vi "UHR-Fleezers Control (host) - Avogadro v3.vi"() -> ()   [LabVIEW 2014] (continued)
  out "Fluorescence laser intensities plot":cluster{dbl, dbl, dbl}(graph)
  in  "Green FB On/Off":bool
  in  "Red FB On/Off":bool
  in  "Blue FB On/Off":bool
  in  "Red Intensity % (FB OFF)":dbl=20.0 min=0.0 max=100.0 step=1.0
  in  "Blue Intensity % (FB OFF)":dbl=87.0 min=0.0 max=100.0 step=1.0
  out "Green laser intensity (V)":dbl
  in  "Initial Phase Adjustment (Green FB)":i16=-30
  in  "Phase adj. (Green FB)":i16=10
  out "Green AI Count":u16=600
  in  "- phase (Green FB)":bool
  in  "+ phase (Green FB)":bool
  out "Relative phase (Green FB)":i16
  out "GI Late Counter 2":u8
  in  "Phase adj. (GI) 2":i16=1
  out "GI relative phase 2":i16
  in  "+ phase (GI) 2":bool
  in  "Initial Phase Adjustment (GI) 2":i16=-274
  in  "- phase (GI) 2":bool
  in  "Green FB Gains":T18={"proportional gain (Kc)"=10, "integral gain (Kc*Ts/Ti)"=5, "derivative gain (Kc*Td/Ts)"=0}
  in  "Green int current ON count adj":u32=150
  out "Green AI Late Counter":u8
  out "MCL Scan":cluster{"Begin (V)":dbl, dbl, dbl[]}(graph)
  out "MCL Scan 2":cluster{"Begin (V)":dbl, dbl, dbl[]}(graph)
  out "Red laser intensity (V)":dbl
  out "Red AI Count":u16=600
  in  "Initial Phase Adjustment (RI)":i16=25
  out "RI Late Counter":u8
  in  "Red FB Gains":T18={"proportional gain (Kc)"=10, "integral gain (Kc*Ts/Ti)"=5, "derivative gain (Kc*Td/Ts)"=0}
  in  "Phase adj. (RI)":i16=20
  out "RI relative phase":i16
  in  "+ phase (RI)":bool
  in  "- phase (RI)":bool
  in  "Blue Laser Modulation Mode":string(combo)
  out "Digital Modulation":bool
  out "Analog Modulation":bool
  out "Laser On":bool
  in  "Get Blue Laser State":bool
  out "Blue laser intensity (V)":dbl
  out "Relative phase (BI AO)":i16
  out "Relative phase (BI DO)":i16
  out "Late Counter (BI DO)":u8
  out "Late Counter (BI AO)":u8
  in  "Initial Phase Adjustment (BI DO)":i16=65
  in  "Initial Phase Adjustment (BI AO)":i16
  in  "Phase adj. (BI AO)":i16=20
  in  "+ phase (BI AO)":bool
  in  "- phase (BI AO)":bool
  in  "Blue int AO ON count adjust":u16=150
  in  "Blue FB Gains":T18={"proportional gain (Kc)"=10, "integral gain (Kc*Ts/Ti)"=5, "derivative gain (Kc*Td/Ts)"=0}
  in  "- phase (BI DO)":bool
  in  "+ phase (BI DO)":bool
  in  "Phase adj. (BI DO)":i16=20
  out "Blue AI Count":u16=600
  in  "Delay (ms)":i32=500
  in  "Send string\nto Blue Laser":bool
  in  "command string":string
  out "command string sent":string="sames 0"
  out "read blue buffer":string
  out "Blue Error Out":errorcluster={"status"=TRUE, "code"=-1073807346, "source"="VISA Write in serial write macro.vi->UHR-Fleezers Control (host) - Avogadro v2.vi"}
  in  "VISA resource name":refnum<visa-resource-name>="Blue-Laser-COM7"
  in  "Blue Laser Modulation\nPower (mW)":string="80"
  in  "Blue Laser Power (mW)\n(Constant Power Mode)":string="70"
  in  "Laser choice 2":enum8{"Blue", "Green", "Red"}(ring)
  in  "Laser choice 1":enum8{"Blue", "Green", "Red"}(ring)
  in  "Laser choice 0":enum8{"Blue", "Green", "Red"}(ring)
  in  "FL interlace OFF count 2":u16=450
  in  "FL interlace OFF count 1":u16=450
  in  "FL interlace OFF count 0":u16=450
  in  "FL interlace ON count 2":u16=150
  in  "Fl interlace ON count 1":u16=150
  in  "FL interlace ON count 0":u16=150
  out "Vortran Late Counter":u8
  in  "Phase adj. (Vortran)":i16=1
  out "Vortran relative phase":i16
  in  "+ phase (Vortran)":bool
  in  "Initial Phase Adjustment (Vortran)":i16=-31
  in  "- phase (Vortran)":bool
  in  "Flip X Sign":bool=TRUE
  in  "Trap Position FIFO Depth":u32=500000 format="%.0p"
  in  "# Samples/trap":u32=20000
  out "Trap AI Elements/DMA read":u32=320000 format="%.0p"
  out "Ave. Rate (Hz)":dbl=200000.0 format="%#_6p"
  out "FIFO El. Rem.":u32=3 format="%.0p"
  in  "Phase adj. (AI1)":i16=10
  out "Relative phase (AI1)":i16=-186
  in  "+ phase (AI1)":bool
  in  "- phase (AI1)":bool
  out "Late Counter (AI1)":u8
  in  "Initial Phase Adjustment (AI1)":i16=186
  out "AI rate (Hz)":dbl=200000.0 format="%#_6p"
  in  "AI Count (ticks)":u16=200
  out "# Samples/channel":u32=40000 format="%.0p"
  in  "Trap AI FIFO Depth":u32=900000
  in  "Detector Type":string(combo)="IR-QPD + PSD + FB-QPD X position"
  in  "N Acq Sets (Traps + Fl.)":i16=2
  in  "Sets to FIFO (Traps)":T26={"Set 1"=TRUE, "Set 2"=TRUE, "Set 3"=FALSE}
  in  "FPGA Ave.":dbl=1.0 min=1.0 step=1.0
  out "Ave. Period (s)":dbl=5e-06 format="%#_6p"
  out "DMA Update Period (s)":dbl=0.2
  out "FPGA Averaging":bool
  out "Trap Sets":u32=2
  out "Counts/DMA":dbl=8000000.0 format="%#_6p"
  out "Trap Pos FIFO El Remaining":u32=17275 format="%.0p"
  out "Trap Pos Elements/DMA read":u32=200000 format="%.0p"
  out "Trap AI FIFO Timeout":u16
  out "Trap Pos FIFO Timeout":u16
  out "error out":errorcluster
  out "error out 2":errorcluster
  in  "Piezo X at\n Scan position (V)":dbl=5.03
  in  "Piezo trap y\noffset (V)":dbl=1.34
  out "Piezo trap x\noffset (V)":dbl=-6.356
  in  "Piezo Trap Y cal (nm/V)":dbl=-289.7
  in  "Piezo Trap X cal (nm/V)":dbl=360.07
  in  "Bottom  1 Harvard Syringe Pump Serial Port":refnum<visa-resource-name>="Bottom-Pump1-COM5"
  in  "Center Harvard Syringe Pump Serial Port":refnum<visa-resource-name>="Central-Pump2-COM6"
  in  "Lost Tether Alarm Threshold (pN)":dbl=0.5
  in  "AOM X Cal (nm/MHz)":dbl=203.0
  in  "MCL X Cal (nm/V)":dbl=739.5
  out "X RF Amplitude Limits (%)":T27={"Minimum"=0.0, "Maximum"=50.0, "Increment"=1.0}
  out "X RF Frequency Limits (MHz)":T27={"Minimum"=60.0, "Maximum"=90.0, "Increment"=1.0}
  out "Y RF Frequency Limits (MHz)":T27={"Minimum"=0.0, "Maximum"=40.0, "Increment"=0.1}
  out "Y RF Amplitude Limits (%)":T27={"Minimum"=0.0, "Maximum"=45.0, "Increment"=1.0}
  in  "Manip. X?":bool=TRUE
  in  "Manip. Y?":bool
  in  "Force Manip Abort":bool
  out "Read cal error":errorcluster
  in  "DAQ Delay (ms)":u32=1000
  in  "Start Scan":bool
  in  "Scan axis":bool=TRUE
  in  "Osc. amp. (V)":dbl=5.0
  in  "Osc. center (V)":dbl=5.0
  in  "Osc. freq. (Hz) 2":dbl=1.0
  in  "MCL Mode":u16(ring) items=["Manual Positioning", "Sinusoidal Wave", "Linear Scan"]
  in  "Begin (V)":dbl
  in  "End (V)":dbl=10.0
  in  "N Points":dbl=20.0
  in  "Delay to Interlace (s)":dbl
  in  "Delayed Interlace Start":bool
  in  "Read Lateness and Rel Phase":bool=TRUE
  out "Vec Mean of T1 T2":dbl[](array[numeric])=[-0.7774650412077682, -0.7721679058471924]
  in  "Cal read wait (s)":u32=5
  out "Time tether formed":timestamp=timestamp(3534521622.0325327 s since 1904-01-01)
  in  "Sample Chamber Stage Serial Port":refnum<visa-resource-name>="Sample-Stage-COM1"
  in  "Chemyx Syringe Pump Serial Port":refnum<visa-resource-name>="ASRL3::INSTR"
  in  "Limit Min (MHz)":dbl=10.0 caption="Min (MHz)"
  in  "Limit Max (MHz)":dbl=16.0 caption="Max (MHz)"
  in  "Limits Enable":bool=TRUE caption="Enable"
  out "AI labels":string[](array[string])=["T1 Y", "T1 X", "T1 Sum", "T2 Y", "T2 X", "T2 Sum", "T1 FB X", "T1 FB Sum", "T2 FB X", "T2 FB Sum", "T3 Y/ PSD Y", "T3 X / PSD X", "T3 Sum / PSD sum"]
  in  "Save Trap Pos. Data":bool=TRUE
  in  "Lower Ch. Cap.":bool
  in  "Top 3 Harvard Syringe Pump Serial Port":refnum<visa-resource-name>="Top-Pump3-COM4"
  out "Database link":path=path "C:/Home/Bustamante Lab/Comstock-LabView-Link.udl"
  out "connection reference":T28
  out "FPGA error out":errorcluster
  out "Trigger Signal":dbl[](graph)=[1.953852737276498, 1.8613052147403675]
  in  "Fish mask thresh":dbl=0.5
  in  "Normal (on) or masked test (off)":bool=TRUE
  in  "Stop F (pN) (mask)":dbl=1.0
  in  "Osc. freq. (Hz)":dbl=0.25
  in  "Trap shift\nmethod":bool=TRUE
  in  "Pause rotation":bool
  out "Waveform Chart":dbl(graph)
  in  "Trap 2 phase shift (deg)":dbl caption="Fixed phase shift (deg)"
  in  "Radius (MHz)":dbl=2.0 min=0.0 max=10.0 step=0.1
  out "Trap trajectories":cluster{dbl[], dbl[]}[](graph)
  in  "Move in a Circle":bool
  in  "Center Y Frequency (MHz)":dbl=31.0
  in  "Stop Moving":bool
  in  "2D Motion Frequency (Hz)":dbl=0.25
  in  "2D Motion Trap Separation (MHz)":dbl=0.75 caption="Fixed distance (MHz)" min=0.0 max=10.0 step=0.1
  in  "Time step (ms)":i64=10
  in  "N steps then stop":i32
  in  "Back to start on finish?":bool=TRUE
  in  "Counterclockwise/Clockwise":bool
  out "Trap 1 sum mean":dbl=-0.03042956290579904 format="%0.2f"
  out "Trap 2 sum mean":dbl=0.02092688161998947 format="%0.2f"
  in  "index 1":i32=3
  in  "index 2":i32
  in  "test":bool
  in  "Reset graph":bool
  in  "N steps to plot":i32=1000
  out "Waveform Graph 2":waveform(dbl)(graph)
  in  "Offset 2":dbl
  in  "mult x":dbl
  in  "Offset":dbl
  out "N data samples":dbl
  out "Initial buffer time (s)":dbl
  in  "N initial buffer elements":u16=5000
  in  "Sound ON":bool
  in  "Carrier Frequency (Hz)":dbl=300.0
  in  "number of samples/ch":i32=100000
  in  "sample mode":T29=1 items=["Finite Samples", "Continuous Samples"]
  in  "device ID":u32
  in  "sound format":T30={"sample rate (S/s)"=22050.0, "number of channels"=2, "bits per sample"=16}
  in  "Volume":dbl=1.0 format="%0.2p"
  in  "interpolation mode":u16(ring)=1 items=["coerce", "linear", "spline", "FIR filter"]
  in  "tone or data":bool
  in  "Data channel to sound":i32
  out "Raw offsets":dbl[](array[numeric])
  out "Trap position array":dbl[](array[numeric])
  out "Multi-MCL offset array":T31(array[cluster])
  in  "Base N trap periods":u32=50
  in  "Period scale factor":dbl=4.0
  in  "Trap osc amp (MHz)":dbl=1.0
  in  "Osc trap cont.":bool
  in  "Osc traps":bool
  out "Trap OSC Period (s)":dbl=0.002
  out "Writing waveform to fpga memory":bool
  in  "Save trap pos with cal":bool=TRUE
  in  "T1 Osc Enable":bool=TRUE
  in  "T2 Osc Enable":bool=TRUE
  out "DMA remainder":u64
  out "(total save/100) /osc period remainder":u32
  out "Total save/100 remainder":u32
  out "N osc/ (total save/100)":u64=25
  out "N osc / DMA":u64=100
  out "N trap osc periods per save":u64
  out "N trap osc periods per save remainder":u64
  in  "Offset file step size":dbl=0.1
  in  "Two Trap Offset Values":T32={"Trap 1X offset"=array[300 elements], "Trap 2X offset"=array[300 elements]}
  in  "Command":string
  out "Reply":string
  in  "Send Command":bool
  out "Preamp Error Out":errorcluster
  in  "Gain Mode":string(combo)="0"
  in  "Invert Signal":bool
  in  "Sensitivity":string(combo)="0"
  in  "Offset Current Sign":bool=TRUE
  in  "Offset Current Value":string(combo)
  in  "Offset Current":bool
  in  "Bias Voltage":bool
  in  "Bias Voltage (mV)":i32
  in  "Filter Type":string(combo)="4"
  in  "Lowpass 3dB Point":string(combo)="6"
  in  "Highpass 3dB Point":string(combo)
  in  "Filter Reset":bool
  out "Command Sent":string
  out "Gain":string(combo)="0"
  # "External fluorescence triggering tests:"
  # "After"
  # "During"
  # "Trap On?"
  # "BD Flow ON?"
  # "Samp Flow ON?"
  # "Trap Trig. Fl.?"
  # "Zero It"
  # "Floor it\n(e.g., hp unwinding)"
  # "1"
  # "2"
  # "Fl. Down"
  # "Fl. Up"
  # "T1 Y"
  # "T1 X"
  # "T1 Sum"
  # "T2 Y"
  # "T2 X"
  # "T2 Sum"
  # "FB1 X"
  # "FB1 Sum"
  # "FB2 X"
  # "FB2 Sum"
  # "T3 Y"
  # "T3 X"
  # "T3 Sum"
  # "Trap Display:"
  # "APD Display:"
  # "2D forces"
  # "Tether lengths"
  # "Tether forces"
  # "Before scanning:\n\nTrap 2 OFF\n\nTraps 1 and 3 ON around same location\n\nTrap ONE bead"
  # "DAQ"
  # "Trap Manipulation"
  # "Bead Calibration"
  # "MCL trap"
  # "Trap 3"
  # "Fl"
  # "Fine Motor Control"
  # "Bottom Pump (#1)"
  # "Central Sample Channels"
  # "Top Pump (#3)"
  # "Rate param is ul/h\nVolume param is ul"
  # "Chemyx Pump 2"
  # "Units: \n1 = ml/m\n2 = ml/h\n3 = ul/m\n4 = ul/h"
  # "Oscillate Set 1 freq. (debugging)"
  # "Some timing delay counts"
  # "If using 2nd RF synth board to control green:\nThen small change in FPGA code to make sets 1 and 2\ncorrespond always to board F1 and F2 so green\ndigital out switches between set 1 and 2 frequencies. \nNo third period. \nSet freq for sets 1 and 3 is zero, set 2 is 80 MHz.\nSet amplitude of all three sets to the same value - no feedback yet."
  # "BD 1"
  # "BD 2"
  # "Trap interlacing RF phase control"
  # "Phase control methods:\n0 = no phase control\n1 = offset increments each trap cycle by values below\n2 = offset increment increases by increment factor each cycle\n3 = random phase (no parameters to set)"
  # "X"
  # "Y"
  # "Only runs at startup. As of 161102, 30% out gives saturated max AOM out. Amp control is 12 bits, so this max corresponds to ~1300."
  # "RG: not sure this actually works - \nwill require wiring changes"
  # "14-bit phase number, i.e., 0 to 16383 (2^14) covers full 2*pi phase."
  # "AOD Raster Scan"
  # "Approx. trap separations"
  # "X"
  # "Y"
  # "FPGA\nreading"
  # "DMA\ntransfer"
  # "APD Integration Loop"
  # "APD Gates"
  # "APD 2 (Cy5)"
  # "APD 3 (Cy2)"
  # "APD 1 (Cy3)"
  # "X"
  # "2D"
  # "Y"
  # "1D"
  # "Analog Out Control (Feedback Loop)"
  # "Laser Intensity Analog Input"
  # "Operational note:\n\nUse the digital out control to adjust red laser\ntiming (fine tuning).\n\nAt the moment, the red laser analog out\ncontrol timing is identical and set by green \nlaser AO timing (in the same loop).  Otherwise\nyou can not get synchronous timing with the\ncurrent AO expansion board.\n\nSimilarly, the AI measurement is also \nsimultaneous for all three lasers (for the same\nreason).\n\nThese controls are kept for possible future\nuse."
  # "Analog Out Control (Feedback Loop)"
  # "Digital Out Control"
  # "Laser Intensity Analog Input"
  # "Operational note:\n\nThe AI measurement is simultaneous for all three lasers\n(see red laser note).\n\nThese controls are kept for possible future use."
  # "Analog Out Control (Feedback Loop)"
  # "Laser Intensity Analog Input"
  # "Digital Out Control"
  # "Gating of Vortran laser"
  # "Digital Out Control"
  # "Total AI Rates (NOT rates/trap)"
  # "(Samples/trap x Trap Sets)"
  # "(Samples/channel x\n8 if averaging (8 channels)\n4 if no averaging)"
  # "Trap 1"
  # "Trap 2"
  # "Flour./Trap 3"
  # "External Video Window"
  # "3: IR LED\n2: Blue LED"
  # "MCL Position Debugging"
  # "Temporary Control Storage\n(these used to be somewhere else, still want to keep them)"
  # "Database config"
  # "Y"
  # "X"
  # "Trap Position Difference Limits"
  # "Start trapping above center (> center MHz)\n\nNegative trap separation means trap 2 follows\n(starts to the right)"
  # "Initialization"
  # "Radius initially determined by center\nand current location (then can be changed)"
  # "Active (oscillating) trap calibration:"
  # "All these remainders\nshould be 0."
  # "DeltaF"
  # "Piezo X"
  # "Piezo Y"
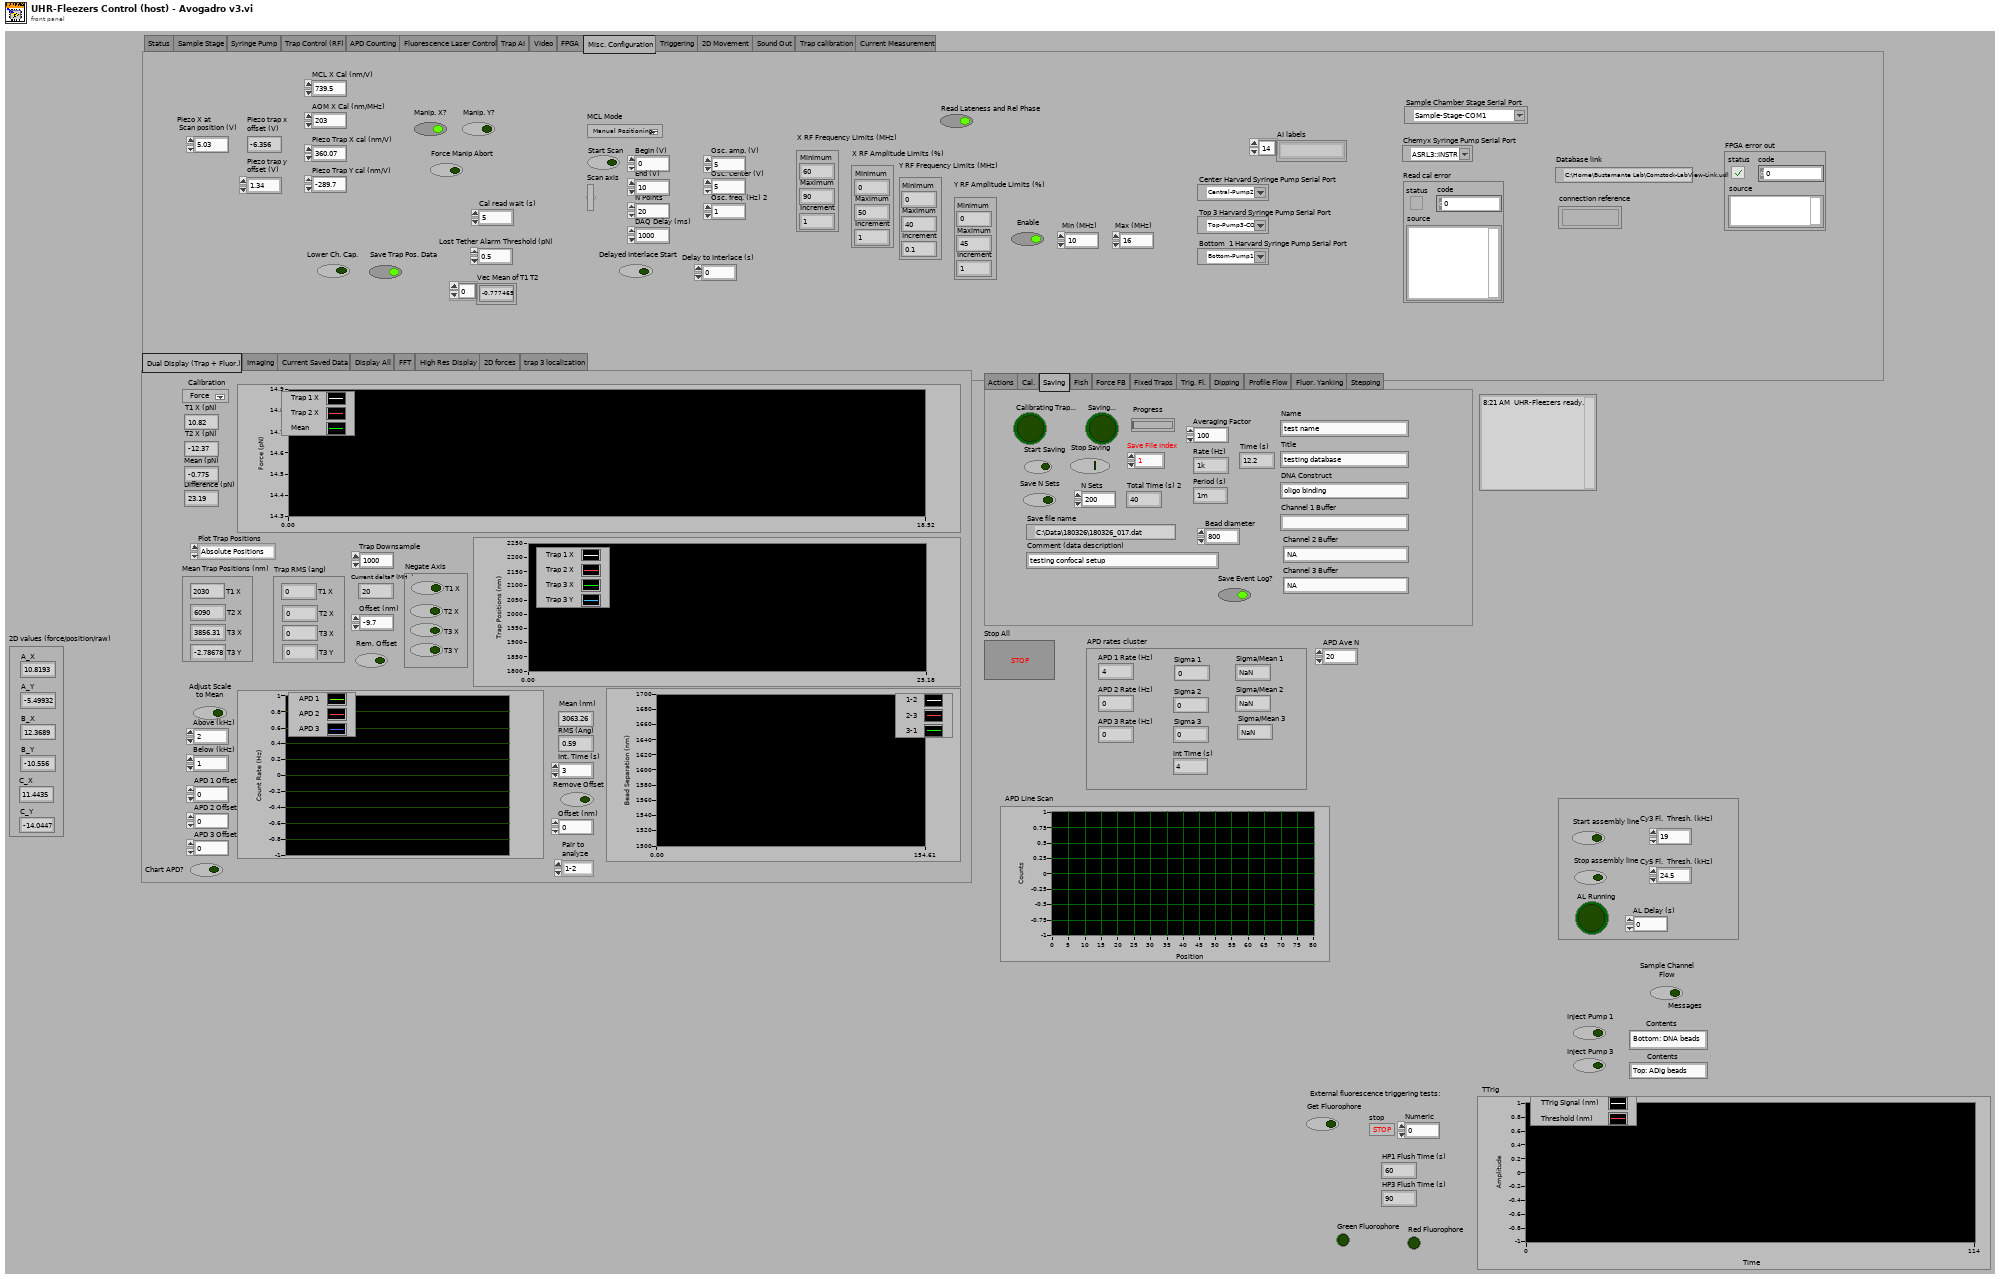
[diagram p1: front panel]
types:
  T1 = cluster{"A_X":dbl, "A_Y":dbl, "B_X":dbl, "B_Y":dbl, "C_X":dbl, "C_Y":dbl}
  T2 = cluster{"APD 1 Rate (Hz)":dbl, "APD 2 Rate (Hz)":dbl, "APD 3 Rate (Hz)":dbl, "Sigma/Mean 1":dbl, "Int Time (s)":dbl, "Sigma 1":dbl, "Sigma 2":dbl, "Sigma 3":dbl, "Sigma/Mean 2":dbl, "Sigma/Mean 3":dbl}
  T3 = enum32{"Actions", "Cal.", "Saving", "Fish", "Force FB", "Fixed Traps", "Trig. Fl.", "Dipping", "Profile Flow", "Fluor. Yanking", "Stepping"}
  T4 = cluster{"Min X":dbl, "Max X":dbl, "Min Y":dbl, "Max Y":dbl, "Scan increment":dbl}
  T5 = enum32{"Dual Display (Trap + Fluor.)", "Imaging", "Current Saved Data", "Display All", "FFT", "High Res Display", "2D forces", "trap 3 localization"}
  T6 = cluster{"T1 X":dbl, "T2 X":dbl, "T3 X":dbl, "T3 Y":dbl}
  T7 = cluster{"T1 X":bool, "T2 X":bool, "T3 X":bool, "T3 Y":bool}
  T8 = typedef "IMAQ Image.ctl" = refnum<image>
  T9 = cluster{"Ext1 (nm)":dbl, "F1 pN)":dbl, "Ext 2 (nm)":dbl, "F2 (pN)":dbl, "Ext 3 (nm)":dbl, "Numeric 6":dbl}
  T10 = cluster{"Xmin":dbl, "Xmax":dbl, "Ymin":dbl, "Ymax":dbl, "increment":dbl}
  T11 = enum32{"Status", "Sample Stage", "Syringe Pump", "Trap Control (RF)", "APD Counting", "Fluorescence Laser Control", "Trap AI", "Video", "FPGA", "Misc. Configuration", "Triggering", "2D Movement", "Sound Out", "Trap calibration", "Current Measurement"}
  T12 = cluster{"alpha_x (nm/V)":dbl, "offset_x (mV)":dbl, "kappa_x (pN/nm)":dbl, "alpha_y (nm/V)":dbl, "kappa_y (pN/nm)":dbl, "offset_y (mV)":dbl}
  T13 = enum32{"Scripts for Shunt ", "Harvard Pumps", "Chemyx Pumps"}
  T14 = cluster{"Pump 1":cluster{"Diameter (mm)":dbl, "Units":dbl, "Volume":dbl, "Rate":dbl}, "Pump 2":cluster{"Diameter (mm)":dbl, "Units":dbl, "Volume":dbl, "Rate":dbl}, "Pump 3":cluster{"Diameter (mm)":dbl, "Units":dbl, "Volume":dbl, "Rate":dbl}}
  T15 = enum32{"IR Laser Interlacing (Direct RF Board Control Method)", "AOD Raster Scan", "Feedback on Trap Intensity", "Feedback on Trap Position"}
  T16 = typedef "LVPoint32TypeDef.ctl" = cluster{"Horizontal":i32, "Vertical":i32}
  T17 = cluster{"Scan Range AOD (nm) 2":dbl, "Step Size AOD (nm) 2":dbl, "Scan Speed AOD (nm/s) 2":dbl, "Number of scans (AOD) 2":u16, "Label":string}[]
  T18 = cluster{"proportional gain (Kc)":i16, "integral gain (Kc*Ts/Ti)":i16, "derivative gain (Kc*Td/Ts)":i16}
  T19 = cluster{"Trap 1":fxp<+/-,16,1>, "Trap 2":fxp<+/-,16,1>}
  T20 = enum32{"Main Setting", "Details", "Dynamic FB settings", "Semi Passive Mode"}
  T21 = cluster{"proportional gain (Kc)":fxp<+/-,16,8>, "integral gain (Kc*Ts/Ti)":fxp<+/-,16,8>, "derivative gain (Kc*Td/Ts)":fxp<+/-,16,8>}
  T22 = cluster{"output high":fxp<+/-,16,1>, "output low":fxp<+/-,16,1>}
  T23 = cluster{"Set 1":fxp<+/-,16,1>, "Set 2":fxp<+/-,16,1>}
  T24 = enum32{"Timing", "MCL Scan", "Analog Out", "EMCCD gating"}
  T25 = enum32{"Main Controls", "Green laser (532 nm)", "Red laser (633 nm)", "Blue laser (473 nm)", "Vortran multi laser"}
  T26 = cluster{"Set 1":bool, "Set 2":bool, "Set 3":bool}
  T27 = typedef "LVMinMaxIncTypeDef.ctl" = cluster{"Minimum":dbl, "Maximum":dbl, "Increment":dbl}
  T28 = typedef "NI_Database_API.lvlib/Conn ObjectReference.ctl" = refnum<k1>
  T29 = typedef "Sampling Mode.ctl" = i32
  T30 = typedef "Sound Data Format.ctl" = cluster{"sample rate (S/s)":dbl, "number of channels":i32, "bits per sample":i32}
  T31 = cluster{"A_X":dbl[], "A_Y":dbl[], "B_X":dbl[], "B_Y":dbl[], "C_X":dbl[], "C_Y":dbl[]}[][]
  T32 = cluster{"Trap 1X offset":dbl[], "Trap 2X offset":dbl[]}
  T33 = typedef "Image Type" = u32
  T34 = typedef "Pressure Control.lvclass/Pressure Control Config.ctl" = cluster{"daqmx_channel":string, "terminal_configuration":string}
  T35 = cluster{string, "TTL line # Pressure Up":u8, bool, bool}
  T36 = cluster{string, "TTL line # Pressure Down":u8, bool, bool}
  T37 = cluster{string, "TTL line # Pressure Vacuum":u8, bool, bool}
  T38 = cluster{string, "TTL line # Pressure Vacuum":u8, bool, bool}[]
  T39 = typedef "nirio_resource_hc.ctl" = tag
  T40 = typedef "openfpgaref.initrf.ctl" = refnum<k20>
  T41 = typedef "openfpgaref.8.6.ctl" = refnum<k20>
  T42 = cluster{"New Image":T8, "New Image":T8, "New Image":T8, "New Image":T8, "New Image":T8}
  T43 = typedef "XDNodeRunTimeDep.lvlib/timing_clust.ctl" = cluster{"Expected End [f-1]":u64, "Actual End [f-1]":u64, "Finished Late? [f-1]":bool, "Expected End [i-1]":u64, "Actual End [i-1]":u64, "Finished Late? [i-1]":bool, "Expected Start [i]":u64, "Actual Start [i]":u64, "Expected Start [f]":u64, "Actual Start [f]":u64, "Source Name":string, "Structure Name":string, "Period":i64, "Deadline":i64, "Offset":i64, "Start":i64, "Priority":i32, "Timeout":i32, "Mode":T44, "Wakeup Reason":T45, "Error":errorcluster, "Source Type":string, "Secondary Source Type":string, "Global End Time":u64, "Global Start Time":u64, "Frame Duration":u64, "Iteration Duration":u64, "Assigned CPU":i32, "I/O Scan Engine Mode":u32}
  T44 = typedef "XDNodeRunTimeDep.lvlib/nitl_modes.ctl" = enum32{"No Change", "Process missed periods, maintain original phase", "Discard missed periods, maintain original phase", "Process missed periods, ignore original phase", "Discard missed periods, ignore original phase"}
  T45 = typedef "XDNodeRunTimeDep.lvlib/wakeup.ctl" = enum32{"Normal", "Aborted", "Asynchronous wakeup", "Timing source error", "Timed loop error", "Timeout"}
  T46 = enum16{"Trackball XY", "Trackball Z", "Trackball OFF", ""}
  T47 = enum32{"Status", "Sample Stage", "Syringe Pump", "Trap Control (RF)", "APD Counting", "Fluorescence Laser Control", "Trap AI", "Video", "FPGA"}
  T48 = enum32{"Status", "Sample Stage", "Syringe Pump", "Trap Control (RF)", "APD Counting", "Fluorescence Laser Control", "Trap AI", "Video", "FPGA", "Misc. Configuration"}
  T49 = enum16{"CONNECT", "INITIALIZE VALVES", "DISCONNECT", "MOVE VALVE"}
  T50 = enum16{"empty", "write", "read oldest (queue)", "read newest (stack)", "read all"}
  T51 = cluster{dbl[], dbl[], dbl[], dbl[], dbl[], dbl[]}
  T52 = cluster{dbl[], dbl[], dbl[], dbl[], dbl[], dbl[]}[][]
  T53 = enum16{"open", "replace", "create", "open or create", "replace or create", "replace or create with confirmation"}
  T54 = enum16{"big-endian, network order", "native, host order", "little-endian"}
  T55 = cluster{"Scan Range AOD (nm) 2":dbl, "Step Size AOD (nm) 2":dbl, "Scan Speed AOD (nm/s) 2":dbl, "Number of scans (AOD) 2":u16, "Label":string}
  T56 = cluster{"alpha_x (nm/V)":dbl, "offset_x (mV)":dbl, "kappa_x (pN/nm)":dbl, "alpha_y (nm/V)":dbl, "kappa_y (pN/nm)":dbl, "offset_y (mV)":dbl}[]
  T57 = cluster{"[0]":dbl, "[1]":dbl, "[2]":dbl, "[3]":dbl, "[4]":dbl, "[5]":dbl}
  T58 = cluster{"Diameter (mm)":dbl, "Units":dbl, "Volume":dbl, "Rate":dbl}
  T59 = cluster{"Left":i32, "Top":i32, "Width":u32, "Height":u32}
  T60 = cluster{cluster{"Left":i32, "Top":i32, "Width":u32, "Height":u32}}[]
  T61 = typedef "Sound Output Task ID.ctl" = u32
  T62 = enum32{"Normal Display", "Dual Display (APD)", "FFT", "High Res Display"}
  T63 = enum32{"Dual Display (Trap + Fluor.)", "Imaging", "Current Saved Data", "Display All", "FFT", "High Res Display"}
  T64 = cluster{"averaging mode":u16, "weighting mode":u16, "number of averages":u32}
  T65 = cluster{"dB On (F)":bool, "unwrap phase (F)":bool, "convert to degree (F)":bool}
  T66 = cluster{"Scan Range (nm)":dbl, "MCL Step Position Ratio":dbl, "MCL/AOM Scale Tweak":dbl, "MCL X Cal (nm/V)":dbl, "MCL Step Increment (V_int)":dbl, "Total Counts (ticks)":u16, "Scan steps (AOD)":u64, "Cycles/step (AOD)":u64}
  T67 = cluster{"Actual MCL Inc (V)":dbl, "Scan steps (MCL)":u64, "Scan lines (y)":u64, "AO1":dbl, "AO2":dbl}
  T68 = cluster{"Actual MCL Inc (V)":dbl, "Scan steps (MCL)":u64, "Scan lines (y)":u64, "T3 Y (V)":dbl, "T3 X (V)":dbl}
  T69 = cluster{"APD 1":u32[], "APD 2":u32[], "APD 3":u32[]}
  T70 = cluster{"X correlation":dbl, "Y correlation":dbl}
  T71 = cluster{"RMS[0]":dbl, "RMS[1]":dbl, "RMS[2]":dbl, "RMS[3]":dbl}
  T72 = cluster{"Mean [0]":dbl, "Mean [1]":dbl, "Mean [2]":dbl, "Mean [3]":dbl}
  T73 = cluster{"T1 X":dbl, "T2 X":dbl, "Mean":dbl, "Difference":dbl}
  T74 = cluster{"f0":dbl, "df":dbl, "magnitude":dbl[]}[][]
  T75 = cluster{"Comment (data description)":string, "Channel 1 Buffer":string, "Channel 2 Buffer":string, "Channel 3 Buffer":string, "Title":string, "DNA Construct":string, "Bead diameter":dbl, "Name":string}
diagram:
  w11 = 90.0
  w33 = T33 2 items=["Grayscale (U8)", "Grayscale (I16)", "Grayscale (SGL)", "Complex (CSG)", "RGB (U32)", "HSL (U32)", "RGB (U64)", "Grayscale (U16)"] ("Image Type")
  # "Stage controller reference"
  # "X limits"
  # "Amp Lmits"
  # "Freq Limits"
  # "Changed by Ronen - All events relating to activation of the pumps have been disabled: 56, 55, 54, 53, 52, 51, 50, 49, 48, 47, 46, 45, 44, 43, 41, 40"
  # "Harvard Pump control disabled by Hendrik"
  # "Bottom 1 Harvard"
  # "Top 3 Harvard"
  # "Center Harvard"
  n1 = disable-structure shown="Enabled" {
    frame Enabled {
      w102 = FALSE
      # "This Control added by\nRonen to enable direct\nControl of pressure pulse\nlength to enable fine flow\ncontrol"
      # "Start out with all lines set to zero"
      n2 = Format Into String(format string="%s/port0/line5:1, %s/port1/line0:3", "DAQmx Device Name", "DAQmx Device Name") -> (resulting string=w94:string)  [unwired: 2 in, 1 out]
      n3 = Format Into String(format string="%s/ai0", "DAQmx Device Name") -> (resulting string=w92:string)  [unwired: 2 in, 1 out]
      n4 = In Range and Coerce(upper limit=100.0, x="Pulse Duration (0-100 ms)", lower limit=0.0) -> (coerced(x)=w77:dbl)  [unwired: 1 out]
      n5 = Bundle By Name(cluster=T34 {"daqmx_channel"="", "terminal_configuration"=""} ("Pressure Control Config"), "daqmx_channel"=w92, "terminal_configuration"="RSE") -> (w109:T34)
      n6 = To Unsigned Long Integer(number=w77) -> (unsigned 32bit integer=w76:u32)
      n7 = Bundle("Pressure up", "TTL line # Pressure Up"=u8 6, w102, w102) -> (w100:T35)  [unwired: 1 in]
      n8 = Bundle("Pressure down", "TTL line # Pressure Down"=u8 8, w102, w102) -> (w101:T36)  [unwired: 1 in]
      n9 = Bundle("Pressure vacuum", "TTL line # Pressure Vacuum"=u8 7, w102, w102) -> (w99:T37)  [unwired: 1 in]
      n10 = Build Array(w100, w101, w99) -> (w98:T38)
      n11 = call "Initialize.vi"("Pulse duration (ms)"=w76, "TTL Ports"=w94, "TTL in"=refnum<class "TTL.lvclass"> refnum ("TTL.lvclass")) -> ("error out"=w97:errorcluster, "TTL out"=w86:refnum<class "TTL.lvclass">)  [unwired: 7 in]
      n12 = call "Initialize.vi"("TTL Lines"=w98, "error in (no error)"=w97, "TTL"=w86, "Pressure Control Config"=w109, "Pressure Control in"=refnum<class "Pressure Control.lvclass"> refnum ("Pressure Control.lvclass")) -> ("error out"=w114:errorcluster, "Pressure Control out"=w96:refnum<class "Pressure Control.lvclass">)  [unwired: 5 in]
      n13 = call "Get line states.vi"("error in (no error)"=w114, "TTL in"=w86) -> ("error out"=w81:errorcluster, "Current line states"=w82:bool[], "TTL out"=w85:refnum<class "TTL.lvclass">)  [unwired: 7 in]
      n14 = Array Size(array=w82) -> (size(s)=w83:i32)
      n15 = for {
        N: w83 -> [_]
        shift-right: [w120] -> w84
        shift-left: w85 -> [w121]
        shift-right: [w118] -> w115
        shift-left: w81 -> [w119]
        i -> [w117]
        n16 = call "Set line.vi"("error in (no error)"=w119, "Action"=enum16{"Open", "Close", "Toggle"}."Open", "Line number"=w117, "TTL in"=w121) -> ("error out"=w118:errorcluster, "TTL out"=w120:refnum<class "TTL.lvclass">)  [unwired: 6 in]
      }
      n17 = case shown="No Error" w115 {
        selector: w115 -> [_ w175]
        tunnel: w96 -> [w126 _]
        tunnel: w84 -> [w125 _]
        tunnel: [w122 w174] -> w89
        frame No Error {
          n18 = while {
            shift-right: [w134] -> w123
            shift-left: w126 -> [w133]
            shift-right: [w132] -> w124
            shift-left: w125 -> [w131]
            stop <- w129 stop-if-true
            n19 = call "Get pressure.vi"("Pressure Control in"=w133) -> ("Pressure"=→"Pressure":dbl)  [unwired: 7 in, 3 out]
            n20 = event shown="[7] \"Pulse Duration (0-100 ms)\": Value Change" {
              selector: _ -> [_ _ _ _ _ _ _ _]
              dyn-events: _ -> [_ _ _ _ _ _ _ _]
              timeout: 100 -> [_ _ _ _ _ _ _ _]
              tunnel: [w137 w140 w141 w146 w150 w155 w160 w172] -> w134
              tunnel: w133 -> [w137 w140 w142 w147 w151 w156 w161 w173]
              tunnel: [w136 w139 w143 w148 w152 w157 w162 w170] -> w132
              tunnel: w131 -> [w136 w139 w143 w148 w152 w157 w162 w171]
              tunnel: [_ TRUE _ _ _ _ _ _] -> w129
              tunnel: [_ _ w144 w149 w153 w158 w163 w169] -> w128
              event Timeout {
                n21 = event-data() -> ()  [unwired: 1 in, 2 out]
              }
              event "Stop All": Value Change {
                n22 = event-data() -> ()  [unwired: 1 in, 6 out]
              }
              event "Vent pressure": Value Change {
                n23 = event-data() -> ()  [unwired: 1 in, 5 out]
                n24 = call "Vent.vi"("Pressure Control in"=w142) -> ("error out"=w144:errorcluster, "Pressure Control out"=w141:refnum<class "Pressure Control.lvclass">)  [unwired: 9 in]
              }
              event "Vacuum": Value Change {
                n25 = event-data() -> ("NewVal"=w145:bool)  [unwired: 1 in, 4 out]
                n26 = call "Set vacuum.vi"("Vacuum?"=w145, "Pressure Control in"=w147) -> ("error out"=w149:errorcluster, "Pressure Control out"=w146:refnum<class "Pressure Control.lvclass">)  [unwired: 8 in]
              }
              event "Set zero pressure": Value Change {
                n27 = event-data() -> ()  [unwired: 1 in, 5 out]
                n28 = call "Set zero pressure to current pressure.vi"("Pressure Control in"=w151) -> ("error out"=w153:errorcluster, "Pressure Control out"=w150:refnum<class "Pressure Control.lvclass">)  [unwired: 8 in, 1 out]
              }
              event "Pressure Up": Value Change {
                n29 = event-data() -> ()  [unwired: 1 in, 5 out]
                n30 = call "Pressure pulse.vi"("Up or down?"=enum16{"Up", "Down"}."Up", "Pressure Control in"=w156) -> ("error out"=w158:errorcluster, "Pressure Control out"=w155:refnum<class "Pressure Control.lvclass">)  [unwired: 8 in]
              }
              event "Pressure Down": Value Change {
                n31 = event-data() -> ()  [unwired: 1 in, 5 out]
                n32 = call "Pressure pulse.vi"("Up or down?"=enum16{"Up", "Down"}."Down", "Pressure Control in"=w161) -> ("error out"=w163:errorcluster, "Pressure Control out"=w160:refnum<class "Pressure Control.lvclass">)  [unwired: 8 in]
              }
              event "Pulse Duration (0-100 ms)": Value Change {
                # "Event added by Ronen to allow for changes\nin pulse duration as program is running"
                n33 = event-data() -> ()  [unwired: 1 in, 6 out]
                n34 = local read "Pulse Duration (0-100 ms)"() -> (w167:dbl)
                n35 = In Range and Coerce(upper limit=100.0, x=w167, lower limit=0.0) -> (coerced(x)=w165:dbl)  [unwired: 1 out]
                n36 = To Unsigned Long Integer(number=w165) -> (unsigned 32bit integer=w164:u32)
                n37 = call "Change TTL - Ronen.vi"("Pulse Duration (ms)"=w164, "TTL.lvclass"=w171) -> ("error out"=w169:errorcluster, "TTL.lvclass"=w170:refnum<class "TTL.lvclass">)  [unwired: 8 in]
                n38 = call "Update TTL - Ronen.vi"("TTL.lvclass"=w170, "Pressure Control in"=w173) -> ("Pressure Control out"=w172:refnum<class "Pressure Control.lvclass">)  [unwired: 8 in, 1 out]
              }
            }
            n39 = call <vilib>:"Simple Error Handler.vi"("error in (no error)"=w128) -> ()  [unwired: 4 in, 5 out]
          }
          n40 = call "Close.vi"("Pressure Control in"=w123) -> ("error out"=w127:errorcluster)  [unwired: 9 in, 1 out]
          n41 = call "Close.vi"("error in (no error)"=w127, "TTL in"=w124) -> ("error out"=w122:errorcluster)  [unwired: 8 in, 1 out]
        }
        frame Error {
          n42 = call <vilib>:"Simple Error Handler.vi"("error in (no error)"=w175) -> ("error out"=w174:errorcluster)  [unwired: 4 in, 4 out]
        }
      }
      n43 = property on="DAQmx Device Name" class="DAQmxName"("Visible"=FALSE) -> ()  [unwired: 2 in, 2 out]
      n44 = call <vilib>:"Clear Errors.vi"("error in (no error)"=w89) -> ("error out"=w87:errorcluster)  [unwired: 5 in, 1 out]
      n45 = property on="DAQmx Device Name" class="DAQmxName"(error in=w87, "Visible"=TRUE) -> ()  [unwired: 1 in, 2 out]
    }
    frame Disabled {
    }
  }
  n46 = disable-structure shown="Disabled" {
    disable-tunnel: [w202 _] -> w45
    disable-tunnel: [w201 _] -> w44
    disable-tunnel: [w196 _] -> w40
    disable-tunnel: [w195 _] -> w39
    disable-tunnel: [w194 _] -> w38
    disable-tunnel: [w193 _] -> w37
    disable-tunnel: [w190 _] -> w29
    disable-tunnel: [w180 _] -> w14
    disable-tunnel: [w177 _] -> w13
    frame Disabled {
      w179 = u16 20 items=["1.0"=10, "1.5"=15, "2.0"=20] ("stop bits (10: 1 bit)")
      w188 = u16 20 items=["1.0"=10, "1.5"=15, "2.0"=20] ("stop bits (10: 1 bit)")
      w191 = u16 10 items=["1.0"=10, "1.5"=15, "2.0"=20] ("stop bits (10: 1 bit)")
      w197 = u16 20 items=["1.0"=10, "1.5"=15, "2.0"=20] ("stop bits (10: 1 bit)")
      w199 = u16 20 items=["1.0"=10, "1.5"=15, "2.0"=20] ("stop bits (10: 1 bit)")
      w203 = u16 20 items=["1.0"=10, "1.5"=15, "2.0"=20] ("stop bits (10: 1 bit)")
      # "Bottom 1 Harvard"
      # "Top 3 Harvard"
      # "Center Harvard"
      n47 = call-poly "VISA Configure Serial Port"("VISA resource name"=refnum<visa-resource-name> "COM2", "baud rate (9600)"=u32 9600, "stop bits (10: 1 bit)"=w188) -> ("VISA resource name out"=w180:refnum<visa-resource-name>, "error out"=→"Preamp Error Out":errorcluster)  [unwired: 4 in, 7 out]
      n48 = call-poly "VISA Configure Serial Port"("VISA resource name"=refnum<visa-resource-name> "COM2", "baud rate (9600)"=u32 9600, "stop bits (10: 1 bit)"=w179) -> ("VISA resource name out"=w177:refnum<visa-resource-name>)  [unwired: 4 in, 8 out]
      n49 = call-poly "VISA Configure Serial Port"("VISA resource name"=refnum<visa-resource-name> "COM7", "baud rate (9600)"=u32 115200, "stop bits (10: 1 bit)"=w191) -> ("VISA resource name out"=w190:refnum<visa-resource-name>, "error out"=w189:errorcluster)  [unwired: 4 in, 7 out]
      n50 = call-poly "VISA Configure Serial Port"("VISA resource name"=refnum<visa-resource-name> "COM5", "baud rate (9600)"=u32 115200, "stop bits (10: 1 bit)"=w197) -> ("VISA resource name out"=w194:refnum<visa-resource-name>, "error out"=w193:errorcluster)  [unwired: 4 in, 7 out]
      n51 = call-poly "VISA Configure Serial Port"("VISA resource name"=refnum<visa-resource-name> "COM4", "baud rate (9600)"=u32 115200, "stop bits (10: 1 bit)"=w199) -> ("VISA resource name out"=w196:refnum<visa-resource-name>, "error out"=w195:errorcluster)  [unwired: 4 in, 7 out]
      n52 = call-poly "VISA Configure Serial Port"("VISA resource name"=refnum<visa-resource-name> "COM6", "baud rate (9600)"=u32 115200, "stop bits (10: 1 bit)"=w203) -> ("VISA resource name out"=w201:refnum<visa-resource-name>, "error out"=w202:errorcluster)  [unwired: 4 in, 7 out]
      n53 = local write "Blue Error Out"(w189) -> ()
    }
    frame Enabled {
    }
  }
  n54 = flat-sequence {
    tunnel: [w209] -> w2
    tunnel: w2 -> [w215]
    tunnel: [w213] -> w1
    frame #0 {
      w209 = T39 "RIO0" ("resource name")
      # "DAQ card ID"
      # "First run the RF synth board initialization fpga code.\n\nThis fpga code essentially enables communication with the RF board using the automatic udclk setting. After running the host initialization vi, the RF boards are fully setup and ready to interlace using the external udclk control. The next fpga code runs the main interlacing instrument methods.\n\nThis host code should run the init bitfile:\n\n'UHR-FleezersInst_FPGATarget_intitializeRFsyn_v1'"
      n55 = xnode "Open FPGA VI Reference"("resource name"=w209) -> ("FPGA VI Reference Out"=w210:T40)  [unwired: 1 in, 1 out]
      n56 = xnode "Invoke Method"("FPGA VI Reference In"=w210) -> ("FPGA VI Reference Out"=w211:T40, "error out"=w212:errorcluster)  [unwired: 1 in]
      n57 = xnode "Invoke Method"("FPGA VI Reference In"=w211, "error in"=w212) -> ("FPGA VI Reference Out"=w208:T40, "error out"=w207:errorcluster)  [unwired: 1 in]
      n58 = call "Initialize RF boards - with FPGA init only vi v1.vi"("error in"=w207, "FPGA Interface"=w208) -> ("error out"=w206:errorcluster, "FPGA Interface 2"=w205:T40)
      n59 = xnode "Close FPGA VI Reference"("FPGA VI Reference In"=w205, "error in"=w206) -> ()  [unwired: 1 out]
    }
    frame #1 {
      w220 = TRUE ("PMODE")
      # "Have to set parallel mode and read to high again (they default to low in the FPGA code)"
      # "Then switch to the main fpga code to run the instrument (interlacing fpga code).\n\nThis host code should run the bitfile:\n\n'UHR-FleezersInst_FPGATarget_UHR-Fleezers_main_16.2.1_v3'"
      # "Reset the DAQ card."
      n60 = xnode "Open FPGA VI Reference"("resource name"=w215) -> ("FPGA VI Reference Out"=w216:T41, "error out"=w217:errorcluster)  [unwired: 1 in]
      n61 = xnode "Invoke Method"("FPGA VI Reference In"=w216, "error in"=w217) -> ("FPGA VI Reference Out"=w218:T41, "error out"=w219:errorcluster)
      n62 = xnode "Read/Write Control"("FPGA VI Reference In"=w218, "error in"=w219, "PMODE"=w220, "RD"=w220) -> ("FPGA VI Reference Out"=w213:T41, "error out"=→"FPGA error out":errorcluster)
    }
  }
  n63 = call "IMAQ Create"("Image Name"="APD 1 Image", "Image Type"=w33) -> ("New Image"=w50:T8)  [unwired: 3 in, 1 out]
  n64 = call "IMAQ Create"("Image Name"="APD 2 Image", "Image Type"=w33) -> ("New Image"=w49:T8)  [unwired: 3 in, 1 out]
  n65 = call "IMAQ Create"("Image Name"="APD 3 Image", "Image Type"=w33) -> ("New Image"=w32:T8)  [unwired: 3 in, 1 out]
  n66 = call "IMAQ Create"("Image Name"="Det. X Image", "Image Type"=w33) -> ("New Image"=w48:T8)  [unwired: 3 in, 1 out]
  n67 = call "IMAQ Create"("Image Name"="Det. Y Image", "Image Type"=w33) -> ("New Image"=w47:T8)  [unwired: 3 in, 1 out]